vi "Dresden R2R Sputter 03.02.2018 IY24.vi"() -> ()   [LabVIEW 2009] (continued)
                  frame #0 {
                    n3645 = stacked-sequence {
                      frame #0 {
                        n3646 = local write "Pps_code_entry"("PF190=" ("Pps_code_entry")) -> ()
                      }
                      frame #1 {
                        n3647 = Wait (ms)(milliseconds to wait=u32 500) -> ()  [unwired: 1 out]
                      }
                      frame #2 {
                        n3648 = local write "Ppsok"(TRUE ("Ppsok")) -> ()
                      }
                    }
                  }
                  frame #1 {
                    n3649 = stacked-sequence {
                      frame #0 {
                        n3650 = local write "Pps_code_entry"("PF189=" ("Pps_code_entry")) -> ()
                      }
                      frame #1 {
                        n3651 = Wait (ms)(milliseconds to wait=u32 500) -> ()  [unwired: 1 out]
                      }
                      frame #2 {
                        n3652 = local write "Ppsok"(TRUE ("Ppsok")) -> ()
                      }
                    }
                  }
                }
              }
            }
            n3653 = case shown="True" w4784 {
              tunnel: w4788 -> [_ w5137]
              frame #0 {
              }
              frame #1 {
                n3654 = case shown="False" w5137 {
                  frame #0 {
                    n3655 = stacked-sequence {
                      frame #0 {
                        n3656 = local write "Pps_code_entry"("PF220=" ("Pps_code_entry")) -> ()
                      }
                      frame #1 {
                        n3657 = Wait (ms)(milliseconds to wait=u32 500) -> ()  [unwired: 1 out]
                      }
                      frame #2 {
                        n3658 = local write "Ppsok"(TRUE ("Ppsok")) -> ()
                      }
                    }
                  }
                  frame #1 {
                    n3659 = stacked-sequence {
                      frame #0 {
                        n3660 = local write "Pps_code_entry"("PF219=" ("Pps_code_entry")) -> ()
                      }
                      frame #1 {
                        n3661 = Wait (ms)(milliseconds to wait=u32 500) -> ()  [unwired: 1 out]
                      }
                      frame #2 {
                        n3662 = local write "Ppsok"(TRUE ("Ppsok")) -> ()
                      }
                    }
                  }
                }
              }
            }
            n3663 = case shown="True" w4944 {
              tunnel: w4948 -> [_ w5368]
              frame #0 {
              }
              frame #1 {
                n3664 = case shown="True" w5368 {
                  frame #0 {
                    n3665 = stacked-sequence {
                      frame #0 {
                        n3666 = local write "Pps_code_entry"("PF156=" ("Pps_code_entry")) -> ()
                      }
                      frame #1 {
                        n3667 = Wait (ms)(milliseconds to wait=u32 500) -> ()  [unwired: 1 out]
                      }
                      frame #2 {
                        n3668 = local write "Ppsok"(TRUE ("Ppsok")) -> ()
                      }
                    }
                  }
                  frame #1 {
                    n3669 = stacked-sequence {
                      frame #0 {
                        n3670 = local write "Pps_code_entry"("PF155=" ("Pps_code_entry")) -> ()
                      }
                      frame #1 {
                        n3671 = Wait (ms)(milliseconds to wait=u32 500) -> ()  [unwired: 1 out]
                      }
                      frame #2 {
                        n3672 = local write "Ppsok"(TRUE ("Ppsok")) -> ()
                      }
                    }
                  }
                }
              }
            }
            n3673 = case shown="True" w5044 {
              tunnel: w5048 -> [_ w5466]
              frame #0 {
              }
              frame #1 {
                n3674 = case shown="True" w5466 {
                  frame #0 {
                    n3675 = stacked-sequence {
                      frame #0 {
                        n3676 = local write "Pps_code_entry"("PF124=" ("Pps_code_entry")) -> ()
                      }
                      frame #1 {
                        n3677 = Wait (ms)(milliseconds to wait=u32 500) -> ()  [unwired: 1 out]
                      }
                      frame #2 {
                        n3678 = local write "Ppsok"(TRUE ("Ppsok")) -> ()
                      }
                    }
                  }
                  frame #1 {
                    n3679 = stacked-sequence {
                      frame #0 {
                        n3680 = local write "Pps_code_entry"("PF123=" ("Pps_code_entry")) -> ()
                      }
                      frame #1 {
                        n3681 = Wait (ms)(milliseconds to wait=u32 500) -> ()  [unwired: 1 out]
                      }
                      frame #2 {
                        n3682 = local write "Ppsok"(TRUE ("Ppsok")) -> ()
                      }
                    }
                  }
                }
              }
            }
            n3683 = case shown="True" w5053 {
              tunnel: w5049 -> [_ w5473]
              frame #0 {
              }
              frame #1 {
                n3684 = case shown="False" w5473 {
                  frame #0 {
                    n3685 = stacked-sequence {
                      frame #0 {
                        n3686 = local write "Pps_code_entry"("PF122=" ("Pps_code_entry")) -> ()
                      }
                      frame #1 {
                        n3687 = Wait (ms)(milliseconds to wait=u32 500) -> ()  [unwired: 1 out]
                      }
                      frame #2 {
                        n3688 = local write "Ppsok"(TRUE ("Ppsok")) -> ()
                      }
                    }
                  }
                  frame #1 {
                    n3689 = stacked-sequence {
                      frame #0 {
                        n3690 = local write "Pps_code_entry"("PF121=" ("Pps_code_entry")) -> ()
                      }
                      frame #1 {
                        n3691 = Wait (ms)(milliseconds to wait=u32 500) -> ()  [unwired: 1 out]
                      }
                      frame #2 {
                        n3692 = local write "Ppsok"(TRUE ("Ppsok")) -> ()
                      }
                    }
                  }
                }
              }
            }
          }
        }
        n3693 = stacked-sequence {
          frame #0 {
            n3694 = local read "Statue_abort"() -> (w4250:bool)
            n3695 = local read "Semi"() -> (w4246:bool)
            n3696 = feedback #116() -> (w4249:bool)  [unwired: 1 in]
            n3697 = case shown="True" w4250 {
              frame #0 {
              }
              frame #1 {
                n3698 = local write "Semi"(TRUE ("Statue_abort")) -> ()
              }
            }
            n3699 = Boolean To (0,1)(Boolean=w4246) -> (0, 1=w4247:i16)
            n3700 = Boolean To (0,1)(Boolean=w4249) -> (0, 1=w4248:i16)
            n3701 = Greater?(x=w4247, y=w4248) -> (0:w4245:bool)
            n3702 = case shown="True" w4245 {
              frame #0 {
              }
              frame #1 {
                n3703 = property on="Process_flow" class="Str"() -> ("Text.Scroll Position"=w4261:u32)  [unwired: 2 in, 2 out]
                n3704 = Get Date/Time String() -> (date string=w4257:string, time string=w4259:string)  [unwired: 3 in]
                n3705 = local read "Process_flow"() -> (w4252:string)
                n3706 = Add(x=w4261, y=u32 10) -> (x+y=w4262:u32)
                n3707 = Concatenate Strings(w4257, " / " ("string"), w4259) -> (w4256:string)
                n3708 = property on="Process_flow" class="Str"("Text.Scroll Position"=w4262) -> ()  [unwired: 2 in, 2 out]
                n3709 = Concatenate Strings(w4256, "-System was aborted." ("PPSCodeEntry")) -> (w4253:string)
                n3710 = Concatenate Strings(w4252, "\r", w4253) -> (w4251:string)
                n3711 = local write "Process_flow"(w4251) -> ()
              }
            }
          }
        }
        n3712 = case shown="True" "Clear_error" {
          frame #0 {
          }
          frame #1 {
            n3713 = local write "Error Message"("" ("Error Message")) -> ()
          }
        }
        n3714 = stacked-sequence {
          frame #0 {
            w4759 = "." ("string")
            # "Date & Time"
            n3715 = Format Date/Time String(time format string (%c)="%d") -> (date/time string=w4757:string)  [unwired: 2 out]
            n3716 = Format Date/Time String(time format string (%c)="%m") -> (date/time string=w4756:string)  [unwired: 2 out]
            n3717 = Format Date/Time String(time format string (%c)="%Y") -> (date/time string=w4758:string)  [unwired: 2 out]
            n3718 = Format Date/Time String(time format string (%c)="%X") -> (date/time string=w4755:string)  [unwired: 2 in]
            n3719 = Concatenate Strings(w4757, w4759, w4756, w4759, w4758, "     " ("string"), w4755) -> (→"Date_time":string)
          }
        }
        n3720 = stacked-sequence {
          frame #0 {
            n3721 = local read "Ch2_Ch_atm_di"() -> (w4295:bool)
            n3722 = local read "Ch1_Ch_atm_di"() -> (w4296:bool)
            n3723 = local read "Ch2_Pl_atm_di"() -> (w4294:bool)
            n3724 = local read "Ch1_Pl_atm_di"() -> (w4297:bool)
            n3725 = case shown="True" w4295 {
              frame #0 {
              }
              frame #1 {
                n3726 = local write "Ch2_Ch_vbv_do"(FALSE ("Ch1_Pl_atm_do")) -> ()
              }
            }
            n3727 = case shown="True" w4296 {
              frame #0 {
              }
              frame #1 {
                n3728 = local write "Ch1_Ch_vbv_do"(FALSE ("Ch1_Pl_atm_do")) -> ()
              }
            }
            n3729 = case shown="True" w4294 {
              frame #0 {
              }
              frame #1 {
                n3730 = local write "Ch2_Pl_vbv_do"(FALSE ("Ch1_Pl_atm_do")) -> ()
              }
            }
            n3731 = case shown="True" w4297 {
              frame #0 {
              }
              frame #1 {
                n3732 = local write "Ch1_Pl_vbv_do"(FALSE ("Ch1_Pl_atm_do")) -> ()
              }
            }
            n3733 = local read "Ch4_Ch_atm_di"() -> (w4292:bool)
            n3734 = local read "Ch3_Ch_atm_di"() -> (w4291:bool)
            n3735 = local read "Ch4_Pl_atm_di"() -> (w4293:bool)
            n3736 = local read "Ch3_Pl_atm_di"() -> (w4290:bool)
            n3737 = case shown="True" w4292 {
              frame #0 {
              }
              frame #1 {
                n3738 = local write "Ch4_Ch_vbv_do"(FALSE ("Ch1_Pl_atm_do")) -> ()
              }
            }
            n3739 = case shown="True" w4291 {
              frame #0 {
              }
              frame #1 {
                n3740 = local write "Ch3_Ch_vbv_do"(FALSE ("Ch1_Pl_atm_do")) -> ()
              }
            }
            n3741 = case shown="True" w4293 {
              frame #0 {
              }
              frame #1 {
                n3742 = local write "Ch4_Pl_vbv_do"(FALSE ("Ch1_Pl_atm_do")) -> ()
              }
            }
            n3743 = case shown="True" w4290 {
              frame #0 {
              }
              frame #1 {
                n3744 = local write "Ch3_Pl_vbv_do"(FALSE ("Ch1_Pl_atm_do")) -> ()
              }
            }
          }
        }
        n3745 = case shown="True" "Left_Direction" {
          frame #0 {
          }
          frame #1 {
            n3746 = local write "Casette_servo_left_direction_do"(TRUE ("Casette_servo_left_direction_do")) -> ()
          }
        }
        n3747 = case shown="True" "Right_Direction" {
          frame #0 {
          }
          frame #1 {
            n3748 = local write "Casette_servo_left_direction_do"(FALSE ("Casette_servo_left_direction_do")) -> ()
          }
        }
      }
    }
    "Background" <- w1835
  }
  n3749 = call <vilib>:"Read JPEG File.vi"("path to JPEG file"="Background_ch4_front_path") -> ("image data"=w542:T34)  [unwired: 8 in, 2 out]
  n3750 = call <vilib>:"MB Serial Init.vi"("Timeout"=i32? 2000, "Mode"=w22, "Parity"=w20, "Baud Rate"=i32? 9600, "VISA resource name"="Moxa I/O 1") -> ("error out"=w16:errorcluster, "VISA resource name out"=w17:refnum<visa-resource-name>)  [unwired: 2 in, 3 out]
  n3751 = call <vilib>:"Read JPEG File.vi"("path to JPEG file"="Background_ch1_front_path") -> ("image data"=w385:T34)  [unwired: 8 in, 2 out]
  n3752 = call <vilib>:"Read JPEG File.vi"("path to JPEG file"="Background_ch4_top_path") -> ("image data"=w541:T34)  [unwired: 8 in, 2 out]
  n3753 = call <vilib>:"Read JPEG File.vi"("path to JPEG file"="Background_ch1_top_path") -> ("image data"=w386:T34)  [unwired: 8 in, 2 out]
  n3754 = Get Date/Time In Seconds() -> (seconds since 1Jan1904=w9:timestamp)
  n3755 = call <vilib>:"Unflatten Pixmap.vi"("image data"=w542) -> ("24-bit pixmap"=w585:u32[][])  [unwired: 4 in, 6 out]
  n3756 = Random Number (0-1)() -> (number: 0 to 1=w5:dbl)
  n3757 = call <vilib>:"Unflatten Pixmap.vi"("image data"=w385) -> ("24-bit pixmap"=w370:u32[][])  [unwired: 4 in, 6 out]
  n3758 = call <vilib>:"Read JPEG File.vi"("path to JPEG file"="Background_ch3_front_path") -> ("image data"=w503:T34)  [unwired: 8 in, 2 out]
  n3759 = call <vilib>:"Unflatten Pixmap.vi"("image data"=w541) -> ("24-bit pixmap"=w584:u32[][])  [unwired: 4 in, 6 out]
  n3760 = call <vilib>:"Unflatten Pixmap.vi"("image data"=w386) -> ("24-bit pixmap"=w371:u32[][])  [unwired: 4 in, 6 out]
  n3761 = Multiply(x=w5, y=i32? 360 ("milliseconds to wait")) -> (x*y=w3:dbl)
  n3762 = call <vilib>:"Unflatten Pixmap.vi"("image data"=w503) -> ("24-bit pixmap"=w571:u32[][])  [unwired: 4 in, 6 out]
  n3763 = call <vilib>:"Read JPEG File.vi"("path to JPEG file"="Background_ch3_top_path") -> ("image data"=w490:T34)  [unwired: 8 in, 2 out]
  n3764 = Build Path(base path="Gui_ch4_front_path", name or relative path="magnetron on.jpg") -> (appended path=w523:path)
  n3765 = Build Path(base path="Gui_ch4_front_path", name or relative path="gv front open.jpg") -> (appended path=w530:path)
  n3766 = Build Path(base path="Gui_ch4_front_path", name or relative path="gv front failed.jpg") -> (appended path=w529:path)
  n3767 = Build Path(base path="Gui_ch4_front_path", name or relative path="magnetron water cooled on.jpg") -> (appended path=w520:path)
  n3768 = Build Path(base path="Gui_ch4_front_path", name or relative path="magnetron water cooled failed.jpg") -> (appended path=w517:path)
  n3769 = Build Path(base path="Gui_ch1_front_path", name or relative path="magnetron on.jpg") -> (appended path=w404:path)
  n3770 = Build Path(base path="Gui_ch1_front_path", name or relative path="gv front open2.jpg") -> (appended path=w397:path)
  n3771 = Build Path(base path="Gui_ch1_front_path", name or relative path="gv front failled2.jpg") -> (appended path=w398:path)
  n3772 = Build Path(base path="Gui_ch1_front_path", name or relative path="magnetron water cooled on.jpg") -> (appended path=w407:path)
  n3773 = Build Path(base path="Gui_ch4_top_path", name or relative path="bv2 on.jpg") -> (appended path=w313:path)
  n3774 = Build Path(base path="Gui_ch4_top_path", name or relative path="sov on.jpg") -> (appended path=w300:path)
  n3775 = Build Path(base path="Gui_ch1_front_path", name or relative path="magnetron water cooled failed.jpg") -> (appended path=w410:path)
  n3776 = Build Path(base path="Gui_ch4_top_path", name or relative path="bv2 fail.jpg") -> (appended path=w310:path)
  n3777 = Build Path(base path="Gui_ch4_top_path", name or relative path="sov fail.jpg") -> (appended path=w303:path)
  n3778 = Build Path(base path="Gui_ch1_front_path", name or relative path="bv3 fail.jpg") -> (appended path=w106:path)
  n3779 = Build Path(base path="Gui_ch4_front_path", name or relative path="bv2 on.jpg") -> (appended path=w365:path)
  n3780 = Build Path(base path="Gui_ch3_front_path", name or relative path="bv3 fail.jpg") -> (appended path=w149:path)
  n3781 = Build Path(base path="Gui_ch3_front_path", name or relative path="gv front open.jpg") -> (appended path=w473:path)
  n3782 = Build Path(base path="Gui_ch3_front_path", name or relative path="magnetron on.jpg") -> (appended path=w477:path)
  n3783 = Build Path(base path="Gui_ch1_front_path", name or relative path="bv3 on.jpg") -> (appended path=w103:path)
  n3784 = Build Path(base path="Gui_ch4_front_path", name or relative path="chamber front piston open drum failed.jpg") -> (appended path=w537:path)
  n3785 = Build Path(base path="Gui_ch4_front_path", name or relative path="bv2 fail.jpg") -> (appended path=w368:path)
  n3786 = Build Path(base path="Gui_ch3_front_path", name or relative path="chamber front piston open.jpg") -> (appended path=w487:path)
  n3787 = Build Path(base path="Gui_ch3_front_path", name or relative path="gv front failed.jpg") -> (appended path=w474:path)
  n3788 = Build Path(base path="Gui_ch3_front_path", name or relative path="bv3 on.jpg") -> (appended path=w146:path)
  n3789 = Build Path(base path="Gui_ch4_front_path", name or relative path="chamber front piston failed drum open.jpg") -> (appended path=w538:path)
  n3790 = Build Path(base path="Gui_ch4_front_path", name or relative path="chamber front piston open.jpg") -> (appended path=w527:path)
  n3791 = Build Path(base path="Gui_ch3_front_path", name or relative path="chamber front piston open drum failed.jpg") -> (appended path=w499:path)
  n3792 = while {
    shift-right: [w5561] -> _
    shift-left: w2 -> [w5538]
    shift-right: [w5558] -> _
    shift-left: i32? 1 -> [w5549]
    shift-right: [w5551] -> _
    shift-left: data[5B] -> [w5557]
    shift-right: [w5550] -> _
    shift-left: i32? 1 -> [w5555]
    shift-right: [w5547] -> _
    shift-left: data[5B] -> [w5556]
    shift-left: w2 -> [w5537]
    shift-right: [w5553] -> _
    shift-left: w9 -> [w5554]
    shift-right: [w5548] -> _
    shift-left: data[5B] ("array") -> [w5552]
    shift-right: [w5536] -> _
    shift-left: data[5B] -> [w5546]
    shift-right: [w5542] -> _
    shift-left: dbl? 6.85 ("To Left Volt") -> [_]
    shift-left: w2 -> [w5541]
    shift-left: w2 -> [_]
    stop <- w5539 stop-if-true
    n3793 = Divide(x=u32 100 ("millisecond multiple"), y=w5549) -> (x/y=w5559:dbl)
    n3794 = local read "Test_stop"() -> (w5544:bool)
    n3795 = Wait Until Next ms Multiple(millisecond multiple=w5559) -> ()  [unwired: 1 out]
    n3796 = Select(t=Roll_StatusT."Stop" ("Roll Status"), s=w5544, f=w5538) -> (s? t:f=w5545:T1)
    n3797 = case shown="\"Start\"" w5545 {
      tunnel: [Roll_StatusT."Initiate" ("Roll Status") w5594 Roll_StatusT."HomeP" ("Roll Status") w5626 w5659 w5686 w5710 w5781 Roll_StatusT."Initiate" ("Roll Status") Roll_StatusT."Stop" ("Roll Status")] -> w5561
      tunnel: [1 w5593 10 10 10 w5670 w5732 10 1 1] -> w5558
      tunnel: [w5567 "Lap Count" w5613 w5629 w5658 w5667 w5716 w5780 w5808 w5825] -> w5551
      tunnel: w5557 -> [w5567 _ w5613 w5629 w5658 w5683 w5715 w5780 w5808 w5825]
      tunnel: [w5568 "Cycle Sayisi" w5614 w5628 w5657 w5671 w5733 w5765 w5809 w5824] -> w5550
      tunnel: w5556 -> [w5566 w5590 w5612 w5631 w5654 w5677 w5728 w5763 w5807 w5826]
      tunnel: [w5566 w5590 w5612 w5631 w5654 w5678 w5728 w5762 w5807 w5826] -> w5547
      tunnel: w5555 -> [w5568 _ w5614 w5628 w5657 w5671 w5733 w5773 w5809 w5824]
      tunnel: w5537 -> [_ _ _ _ _ _ w5708 _ _ _]
      tunnel: w5554 -> [_ w5588 w5609 _ _ w5676 _ w5772 w5811 w5820]
      tunnel: [w5564 w5588 w5609 w5625 w5655 w5675 w5730 w5771 w5811 w5820] -> w5553
      tunnel: w5552 -> [w5569 w5589 w5610 w5624 w5656 w5672 w5724 w5770 w5812 w5821]
      tunnel: [w5569 w5589 w5610 w5624 w5656 w5673 w5723 w5769 w5813 w5821] -> w5548
      tunnel: w5549 -> [_ _ _ _ _ w5670 w5732 _ _ _]
      tunnel: [w5565 w5583 w5608 w5630 w5651 w5668 w5731 w5766 0 0] -> w5536
      tunnel: w5546 -> [w5565 w5587 w5608 w5630 w5651 w5668 w5731 w5766 _ _]
      tunnel: [w5563 w5584 w5607 w5632 w5649 w5666 w5726 w5761 w5803 w5817] -> w5542
      tunnel: "Speed" -> [w5563 w5584 w5607 w5632 w5649 w5666 w5726 w5761 w5803 w5817]
      tunnel: w5537 -> [_ _ _ _ _ _ w5725 _ _ _]
      tunnel: "Speed" -> [_ _ _ _ _ _ _ _ _ _]
      tunnel: w5541 -> [_ _ _ _ _ _ _ _ _ _]
      frame #0 {
        n3798 = flat-sequence {
          tunnel: [w5579] -> w5562
          tunnel: w5562 -> [w5581]
          frame #0 {
            w5572 = FALSE ("Ch1_Motor_DO")
            n3799 = local write "Ch2_SRV_start_stop_do"(w5572) -> ()
            n3800 = local write "Ch3_SRV_start_stop_do"(w5572) -> ()
            n3801 = local write "Ch4_SRV_start_stop_do"(w5572) -> ()
            n3802 = local write "Ch1_SRV_start_stop_do"(w5572) -> ()
            n3803 = local write "Ch1_Motor_DO"(w5572) -> ()
            n3804 = local write "Ch2_Motor_DO"(w5572) -> ()
            n3805 = local write "Ch3_Motor_DO"(w5572) -> ()
            n3806 = local write "Ch4_Motor_DO"(w5572) -> ()
          }
          frame #1 {
            w5573 = sgl 15.0 ("TC1_set_value")
            n3807 = local write "TC2_set_value"(w5573) -> ()
            n3808 = local write "TC1_set_value"(w5573) -> ()
            n3809 = Wait (ms)(milliseconds to wait=u32 10000) -> ()  [unwired: 1 out]
          }
          frame #2 {
            w5577 = 0.9
            n3810 = local write "To Right Volt"(w5577) -> ()
            n3811 = local write "To Left Volt"(0.9) -> ()
            n3812 = local write "To Left Volt"(w5577) -> ()
            n3813 = local write "TC1_set"(TRUE ("Tension Parametre Set Yolla")) -> ()
          }
          frame #3 {
            w5579 = TRUE ("Tension Parametre Set Yolla")
            n3814 = local write "Parameters_set"(w5579) -> ()
            n3815 = Wait (ms)(milliseconds to wait=u32 10000) -> ()  [unwired: 1 out]
          }
          frame #4 {
            n3816 = local write "Calculate_auto"(w5581) -> ()
            n3817 = Wait (ms)(milliseconds to wait=u32 10000) -> ()  [unwired: 1 out]
          }
        }
        n3818 = Get Date/Time In Seconds() -> (seconds since 1Jan1904=w5564:timestamp)
      }
      frame #1 {
        w5586 = 0.0 ("Forward Time")
        # "Kac metre gidilecek bilgisi alınır\nKac tur atacak bilgisi alınır"
        n3819 = local read "Start_roll"() -> (w5585:bool)
        n3820 = case shown="True" w5585 {
          tunnel: [Roll_StatusT."Initiate" ("Roll Status") w5598] -> w5594
          tunnel: [1 10] -> w5593
          tunnel: w5587 -> [_ w5601]
          frame #0 {
          }
          frame #1 {
            n3821 = Not Equal?(x=w5601, y=0) -> (x != y?=w5599:bool)
            n3822 = Wait (ms)(milliseconds to wait=u32 1000) -> ()  [unwired: 1 out]
            n3823 = Select(t=Roll_StatusT."Start" ("Roll Status"), s=w5599, f=Roll_StatusT."Security" ("Roll Status")) -> (s? t:f=w5598:T1)
          }
        }
        n3824 = local write "Forward Time"(w5586) -> ()
        n3825 = local write "Bacward Time"(w5586) -> ()
        n3826 = local read "ch_present_position"() -> (w5583:dbl)
        n3827 = Decrement(x=w5583) -> (x-1=w5582:dbl)
        n3828 = local write "Target Chamber Sensor"(w5582) -> ()
      }
      frame #2 {
        w5606 = 0.9
        n3829 = case shown="4" w5608 {
          frame #0 {
          }
          frame #1 {
            w5616 = TRUE ("Ch1_Motor_DO")
            n3830 = local write "Ch1_Motor_DO"(w5616) -> ()
            n3831 = local write "Ch1_SRV_start_stop_do"(w5616) -> ()
          }
          frame #2 {
            w5617 = TRUE ("Ch1_Motor_DO")
            n3832 = local write "Ch2_Motor_DO"(w5617) -> ()
            n3833 = local write "Ch2_SRV_start_stop_do"(w5617) -> ()
          }
          frame #3 {
            w5618 = TRUE ("Ch1_Motor_DO")
            n3834 = local write "Ch3_Motor_DO"(w5618) -> ()
            n3835 = local write "Ch3_SRV_start_stop_do"(w5618) -> ()
          }
          frame #4 {
            w5619 = TRUE ("Ch1_Motor_DO")
            n3836 = local write "Ch4_Motor_DO"(w5619) -> ()
            n3837 = local write "Ch4_SRV_start_stop_do"(w5619) -> ()
          }
        }
        n3838 = local write "To Right Volt"(w5606) -> ()
        n3839 = local write "To Left Volt"(0.9) -> ()
        n3840 = local write "To Left Volt"(w5606) -> ()
      }
      frame #3 {
        w5621 = 0.9
        # "Dolu yarim aya girince baslatir."
        n3841 = case shown="1" w5630 {
          tunnel: [FALSE ("Ch4_Sensor_DI") w5639 w5640 w5641 w5642] -> w5635
          frame #0 {
          }
          frame #1 {
            n3842 = local read "Ch1_Sensor_DI"() -> (w5639:bool)
          }
          frame #2 {
            n3843 = local read "Ch2_Sensor_DI"() -> (w5640:bool)
          }
          frame #3 {
            n3844 = local read "Ch3_Sensor_DI"() -> (w5641:bool)
          }
          frame #4 {
            n3845 = local read "Ch4_Sensor_DI"() -> (w5642:bool)
          }
        }
        n3846 = feedback #117(FALSE ("Ch4_Sensor_DI")) -> (w5622:bool)
        n3847 = Not(x=w5635) -> (.not. x?=w5623:bool)
        n3848 = And(x=w5623, y=w5622) -> (x .and. y?=w5637:bool)
        n3849 = local write "To Right Volt"(w5621) -> ()
        n3850 = local write "To Left Volt"(0.9) -> ()
        n3851 = local write "To Left Volt"(w5621) -> ()
        n3852 = Select(t=Roll_StatusT."Pause" ("Roll Status"), s=w5637, f=Roll_StatusT."HomeP" ("Roll Status")) -> (s? t:f=w5626:T1)
        n3853 = Get Date/Time In Seconds() -> (seconds since 1Jan1904=w5625:timestamp)
      }
      frame #4 {
        # "Dolu yarim aya girince baslatir."
        n3854 = case shown="4" w5651 {
          tunnel: [FALSE ("Ch4_Sensor_DI") w5662 w5663 w5664 w5665] -> w5652
          frame #0 {
          }
          frame #1 {
            n3855 = local read "Ch1_Sensor_DI"() -> (w5662:bool)
          }
          frame #2 {
            n3856 = local read "Ch2_Sensor_DI"() -> (w5663:bool)
          }
          frame #3 {
            n3857 = local read "Ch3_Sensor_DI"() -> (w5664:bool)
          }
          frame #4 {
            n3858 = local read "Ch4_Sensor_DI"() -> (w5665:bool)
          }
        }
        n3859 = feedback #118(FALSE ("Ch4_Sensor_DI")) -> (w5645:bool)
        n3860 = Not(x=w5652) -> (.not. x?=w5646:bool)
        n3861 = And(x=w5646, y=w5645) -> (x .and. y?=w5647:bool)
        n3862 = local write "To Left Volt"(0.9) -> ()
        n3863 = local write "To Left Volt"(0.9) -> ()
        n3864 = Select(t=Roll_StatusT."Pause" ("Roll Status"), s=w5647, f=Roll_StatusT."Home" ("Roll Status")) -> (s? t:f=w5659:T1)
        n3865 = Get Date/Time In Seconds() -> (seconds since 1Jan1904=w5655:timestamp)
      }
      frame #5 {
        # "Baslangicta dolu yarim ayda ilerler,\nIlk tur icinde once bosa cikar ve\nDolu yarim aya tekrar girince tur atmis olur."
        # "Turları geriye sarma islemi yapılıyor"
        n3866 = case shown="4" w5668 {
          tunnel: [FALSE ("Ch1_Home_DO") w5691 w5692 w5693 w5694] -> w5669
          frame #0 {
          }
          frame #1 {
            n3867 = local read "Ch1_Sensor_DI"() -> (w5691:bool)
          }
          frame #2 {
            n3868 = local read "Ch2_Sensor_DI"() -> (w5692:bool)
          }
          frame #3 {
            n3869 = local read "Ch3_Sensor_DI"() -> (w5693:bool)
          }
          frame #4 {
            n3870 = local read "Ch4_Sensor_DI"() -> (w5694:bool)
          }
        }
        n3871 = feedback #119(TRUE ("Ch1_Home_DO")) -> (w5689:bool)
        n3872 = Not(x=w5689) -> (.not. x?=w5688:bool)
        n3873 = And(x=w5669, y=w5688) -> (x .and. y?=w5680:bool)
        n3874 = local write "To Left Volt"(w5666) -> ()
        n3875 = local write "To Right Volt"(w5666) -> ()
        n3876 = Increment(x=w5677) -> (x+1=w5679:i32)
        n3877 = Decrement(x=w5683) -> (x-1=w5687:i32)
        n3878 = Select(t=w5679, s=w5680, f=w5677) -> (s? t:f=w5678:i32)
        n3879 = Select(t=w5687, s=w5680, f=w5683) -> (s? t:f=w5667:i32)
        n3880 = Less Or Equal?(x=w5667, y=0) -> (x <= y?=w5674:bool)
        n3881 = Select(t=Roll_StatusT."Pause" ("Roll Status"), s=w5674, f=Roll_StatusT."Forward" ("Roll Status")) -> (s? t:f=w5686:T1)
        n3882 = case shown="False" w5674 {
          tunnel: [w5697 w5702] -> w5675
          tunnel: w5676 -> [w5697 _]
          tunnel: [w5695 w5699] -> w5673
          tunnel: w5672 -> [w5695 w5701]
          frame #0 {
            n3883 = Get Date/Time In Seconds() -> (seconds since 1Jan1904=w5698:timestamp)
            n3884 = Subtract(x=w5698, y=w5697) -> (x-y=→"Forward Time":dbl)
          }
          frame #1 {
            n3885 = local read "Forward Time"() -> (w5700:dbl)
            n3886 = Get Date/Time In Seconds() -> (seconds since 1Jan1904=w5702:timestamp)
            n3887 = Build Array (concatenate)(w5701, w5700) -> (w5699:dbl[])
          }
        }
      }
      frame #6 {
        w5703 = 0.9 ("To Left Volt")
        w5729 = 0.0 ("milliseconds to wait")
        n3888 = flat-sequence {
          tunnel: w5725 -> [w5739]
          tunnel: [w5748] -> w5727
          tunnel: w5727 -> [w5751]
          tunnel: w5731 -> [w5755]
          tunnel: [w5754] -> w5730
          frame #0 {
            w5734 = FALSE ("Ch1_Motor_DO")
            n3889 = local write "Ch2_SRV_start_stop_do"(w5734) -> ()
            n3890 = local write "Ch3_SRV_start_stop_do"(w5734) -> ()
            n3891 = local write "Ch4_SRV_start_stop_do"(w5734) -> ()
            n3892 = local write "Ch1_SRV_start_stop_do"(w5734) -> ()
            n3893 = local write "Ch1_Motor_DO"(w5734) -> ()
            n3894 = local write "Ch2_Motor_DO"(w5734) -> ()
            n3895 = local write "Ch3_Motor_DO"(w5734) -> ()
            n3896 = local write "Ch4_Motor_DO"(w5734) -> ()
            n3897 = local write "Start_roll"(FALSE ("Start")) -> ()
          }
          frame #1 {
            n3898 = Equal?(x=Roll_StatusT."Backward" ("Roll Status"), y=w5739) -> (x = y?=w5740:bool)
            n3899 = Equal?(x=Roll_StatusT."Home" ("Roll Status"), y=w5739) -> (x = y?=w5737:bool)
            n3900 = Or(x=w5737, y=w5740) -> (x .or. y?=w5736:bool)
            n3901 = case shown="False" w5736 {
              frame #0 {
                n3902 = local read "Roll_side_select"() -> (w5744:enum32{"Left to Right", "Right to Left"})
                n3903 = Equal?(x=enum32{"Left to Right", "Right to Left"}."Left to Right" ("Roll_side_select"), y=w5744) -> (x = y?=w5745:bool)
                n3904 = case shown="True" w5745 {
                  frame #0 {
                    n3905 = local write "Roll_side_select"(enum32{"Left to Right", "Right to Left"}."Left to Right" ("Roll_side_select")) -> ()
                  }
                  frame #1 {
                    n3906 = local write "Roll_side_select"(enum32{"Left to Right", "Right to Left"}."Right to Left" ("Roll_side_select")) -> ()
                  }
                }
              }
              frame #1 {
              }
            }
            n3907 = Wait (ms)(milliseconds to wait=u32 1000) -> ()  [unwired: 1 out]
          }
          frame #2 {
            w5748 = TRUE ("Tension Parametre Set Yolla")
            n3908 = local write "Tension Parametre Set"(w5748) -> ()
            n3909 = local write "Parameters_set"(w5748) -> ()
            n3910 = Wait (ms)(milliseconds to wait=u32 5000) -> ()  [unwired: 1 out]
          }
          frame #3 {
            n3911 = local write "Calculate_auto"(w5751) -> ()
            n3912 = Wait (ms)(milliseconds to wait=u32 5000) -> ()  [unwired: 1 out]
          }
          frame #4 {
            n3913 = local write "Start_roll"(TRUE ("Start")) -> ()
            n3914 = Wait (ms)(milliseconds to wait=u32 1000) -> ()  [unwired: 1 out]
          }
          frame #5 {
            n3915 = case shown="4" w5755 {
              frame #0 {
              }
              frame #1 {
                w5756 = TRUE ("Ch1_Motor_DO")
                n3916 = local write "Ch1_SRV_start_stop_do"(w5756) -> ()
                n3917 = local write "Ch1_Motor_DO"(w5756) -> ()
              }
              frame #2 {
                w5757 = TRUE ("Ch1_Motor_DO")
                n3918 = local write "Ch2_SRV_start_stop_do"(w5757) -> ()
                n3919 = local write "Ch2_Motor_DO"(w5757) -> ()
              }
              frame #3 {
                w5758 = TRUE ("Ch1_Motor_DO")
                n3920 = local write "Ch3_SRV_start_stop_do"(w5758) -> ()
                n3921 = local write "Ch3_Motor_DO"(w5758) -> ()
              }
              frame #4 {
                w5759 = TRUE ("Ch1_Motor_DO")
                n3922 = local write "Ch4_SRV_start_stop_do"(w5759) -> ()
                n3923 = local write "Ch4_Motor_DO"(w5759) -> ()
              }
            }
            n3924 = Get Date/Time In Seconds() -> (seconds since 1Jan1904=w5754:timestamp)
          }
        }
        n3925 = Equal?(x=Roll_StatusT."Forward" ("Roll Status"), y=w5708) -> (x = y?=w5717:bool)
        n3926 = Equal?(x=Roll_StatusT."Backward" ("Roll Status"), y=w5708) -> (x = y?=w5707:bool)
        n3927 = Select(t=Roll_StatusT."HomeP" ("Roll Status"), s=w5707, f=Roll_StatusT."Forward" ("Roll Status")) -> (s? t:f=w5705:T1)
        n3928 = local write "To Right Volt"(w5703) -> ()
        n3929 = local write "To Left Volt"(w5703) -> ()
        n3930 = local read "Lap Count"() -> (w5720:i32)
        n3931 = Increment(x=w5720) -> (x+1=w5719:i32)
        n3932 = Select(t=Roll_StatusT."Backward" ("Roll Status"), s=w5717, f=w5705) -> (s? t:f=w5711:T1)
        n3933 = Build Array (concatenate)(w5724, u32 0 ("milliseconds to wait")) -> (w5723:dbl[])
        n3934 = Select(t=w5715, s=w5717, f=w5719) -> (s? t:f=w5716:i32)
        n3935 = local write "Bacward Time"(w5729) -> ()
        n3936 = local write "Forward Time"(w5729) -> ()
        n3937 = Equal?(x=Roll_StatusT."HomeP" ("Roll Status"), y=w5708) -> (x = y?=w5713:bool)
        n3938 = Select(t=Roll_StatusT."Home" ("Roll Status"), s=w5713, f=w5711) -> (s? t:f=w5710:T1)
      }
      frame #7 {
        n3939 = case shown="1" w5766 {
          tunnel: [FALSE ("Ch1_Home_DO") w5789 w5790 w5791 w5792] -> w5767
          frame #0 {
          }
          frame #1 {
            n3940 = local read "Ch1_Sensor_DI"() -> (w5789:bool)
          }
          frame #2 {
            n3941 = local read "Ch2_Sensor_DI"() -> (w5790:bool)
          }
          frame #3 {
            n3942 = local read "Ch3_Sensor_DI"() -> (w5791:bool)
          }
          frame #4 {
            n3943 = local read "Ch4_Sensor_DI"() -> (w5792:bool)
          }
        }
        n3944 = Decrement(x=w5773) -> (x-1=w5779:i32)
        n3945 = feedback #120(TRUE ("Ch1_Home_DO")) -> (w5764:bool)
        n3946 = local write "To Right Volt"(w5761) -> ()
        n3947 = local write "To Left Volt"(w5761) -> ()
        n3948 = Not(x=w5767) -> (.not. x?=w5784:bool)
        n3949 = And(x=w5784, y=w5764) -> (x .and. y?=w5787:bool)
        n3950 = Decrement(x=w5763) -> (x-1=w5786:i32)
        n3951 = Select(t=w5786, s=w5787, f=w5763) -> (s? t:f=w5762:i32)
        n3952 = Less Or Equal?(x=w5762, y=0) -> (x <= y?=w5760:bool)
        n3953 = Select(t=w5779, s=w5760, f=w5773) -> (s? t:f=w5765:i32)
        n3954 = Less Or Equal?(x=w5765, y=0) -> (x <= y?=w5778:bool)
        n3955 = Select(t=Roll_StatusT."Stop" ("Roll Status"), s=w5778, f=Roll_StatusT."Pause" ("Roll Status")) -> (s? t:f=w5774:T1)
        n3956 = Select(t=w5774, s=w5760, f=Roll_StatusT."Backward" ("Roll Status")) -> (s? t:f=w5781:T1)
        n3957 = case shown="True" w5760 {
          tunnel: [w5796 w5801] -> w5771
          tunnel: w5772 -> [w5796 _]
          tunnel: w5770 -> [w5794 w5799]
          tunnel: [w5794 w5800] -> w5769
          frame #0 {
            n3958 = Get Date/Time In Seconds() -> (seconds since 1Jan1904=w5797:timestamp)
            n3959 = Subtract(x=w5797, y=w5796) -> (x-y=w5795:dbl)
            n3960 = Negate(x=w5795) -> (-x=→"Bacward Time":dbl)
          }
          frame #1 {
            n3961 = local read "Bacward Time"() -> (w5798:dbl)
            n3962 = Get Date/Time In Seconds() -> (seconds since 1Jan1904=w5801:timestamp)
            n3963 = Build Array (concatenate)(w5799, w5798) -> (w5800:dbl[])
          }
        }
      }
      frame #8 {
        w5802 = FALSE ("Ch1_Motor_DO")
        n3964 = Wait (ms)(milliseconds to wait=u32 1000) -> ()  [unwired: 1 out]
        n3965 = local write "Start_roll"(FALSE ("Start")) -> ()
        n3966 = local write "Ch1_Motor_DO"(w5802) -> ()
        n3967 = local write "Ch2_Motor_DO"(w5802) -> ()
        n3968 = local write "Ch3_Motor_DO"(w5802) -> ()
        n3969 = local write "Ch4_Motor_DO"(w5802) -> ()
        n3970 = local write "Ch1_SRV_start_stop_do"(w5802) -> ()
        n3971 = local write "Ch2_SRV_start_stop_do"(w5802) -> ()
        n3972 = local write "Ch3_SRV_start_stop_do"(w5802) -> ()
        n3973 = local write "Ch4_SRV_start_stop_do"(w5802) -> ()
        n3974 = Build Array (concatenate)(w5812, u32 0 ("milliseconds to wait")) -> (w5813:dbl[])
      }
      frame #9 {
        w5816 = FALSE ("Ch1_Motor_DO")
        n3975 = local write "Ch1_Motor_DO"(w5816) -> ()
        n3976 = local write "Ch2_Motor_DO"(w5816) -> ()
        n3977 = local write "Ch3_Motor_DO"(w5816) -> ()
        n3978 = local write "Ch4_Motor_DO"(w5816) -> ()
        n3979 = local write "Ch1_SRV_start_stop_do"(w5816) -> ()
        n3980 = local write "Ch2_SRV_start_stop_do"(w5816) -> ()
        n3981 = local write "Ch3_SRV_start_stop_do"(w5816) -> ()
        n3982 = local write "Ch4_SRV_start_stop_do"(w5816) -> ()
        n3983 = local write "Start_roll"(FALSE ("Start")) -> ()
      }
    }
    "Current Forward Lap" <- w5551
    "Current Cycle" <- w5550
    "Lap Times" <- w5548
    "Current Backward Lap" <- w5547
    "Current Chamber" <- w5536
    n3984 = local read "Test_stop"() -> (w5539:bool)
    "Roll Status" <- w5538
  }
  n3985 = Build Path(base path="Gui_ch3_front_path", name or relative path="chamber front piston failed drum open.jpg") -> (appended path=w500:path)
  n3986 = Build Path(base path="Gui_ch3_front_path", name or relative path="magnetron water cooled on.jpg") -> (appended path=w480:path)
  n3987 = Build Path(base path="Gui_ch3_front_path", name or relative path="magnetron water cooled failed.jpg") -> (appended path=w483:path)
  n3988 = Build Path(base path="Gui_ch1_front_path", name or relative path="chamber front piston open drum failed.jpg") -> (appended path=w390:path)
  n3989 = Build Path(base path="Gui_ch1_front_path", name or relative path="chamber front piston failed drum open.jpg") -> (appended path=w389:path)
  n3990 = Build Path(base path="Gui_ch1_front_path", name or relative path="chamber front piston open.jpg") -> (appended path=w400:path)
  n3991 = Build Path(base path="Gui_ch3_front_path", name or relative path="gv front failled2.jpg") -> (appended path=w359:path)
  n3992 = Build Path(base path="Gui_ch3_front_path", name or relative path="gv front open2.jpg") -> (appended path=w356:path)
  n3993 = call <vilib>:"Read JPEG File.vi"("path to JPEG file"="Background_ch2_front_path") -> ("image data"=w463:T34)  [unwired: 8 in, 2 out]
  n3994 = Build Path(base path="Gui_ch2_top_path", name or relative path="bv2 on.jpg") -> (appended path=w276:path)
  n3995 = Build Path(base path="Gui_ch4_top_path", name or relative path="chamber 1 top piston open.jpg") -> (appended path=w512:path)
  n3996 = call <vilib>:"Unflatten Pixmap.vi"("image data"=w490) -> ("24-bit pixmap"=w566:u32[][])  [unwired: 4 in, 6 out]
  n3997 = Build Path(base path="Gui_ch2_top_path", name or relative path="sov on.jpg") -> (appended path=w286:path)
  n3998 = Build Path(base path="Gui_ch4_top_path", name or relative path="chamber 1 top piston failed.jpg") -> (appended path=w511:path)
  n3999 = Build Path(base path="Gui_ch2_top_path", name or relative path="bv2 fail.jpg") -> (appended path=w279:path)
  n4000 = Build Path(base path="Gui_ch4_top_path", name or relative path="atm3 fail.jpg") -> (appended path=w349:path)
  n4001 = Build Path(base path="Gui_ch2_top_path", name or relative path="sov fail.jpg") -> (appended path=w283:path)
  n4002 = Build Path(base path="Gui_ch2_front_path", name or relative path="gv front open.jpg") -> (appended path=w456:path)
  n4003 = Build Path(base path="Gui_ch2_front_path", name or relative path="magnetron on.jpg") -> (appended path=w452:path)
  n4004 = Build Path(base path="Gui_ch4_top_path", name or relative path="atm3 on.jpg") -> (appended path=w348:path)
  n4005 = Build Path(base path="Gui_ch4_top_path", name or relative path="pg2 fail.jpg") -> (appended path=w340:path)
  n4006 = Build Path(base path="Gui_ch4_top_path", name or relative path="cc fail.jpg") -> (appended path=w333:path)
  n4007 = Build Path(base path="Gui_ch4_top_path", name or relative path="pg2 fail.jpg") -> (appended path=w325:path)
  n4008 = Build Path(base path="Gui_ch2_top_path", name or relative path="bv3 fail.jpg") -> (appended path=w155:path)
  n4009 = Build Path(base path="Gui_ch2_front_path", name or relative path="chamber front piston open.jpg") -> (appended path=w444:path)
  n4010 = Build Path(base path="Gui_ch2_front_path", name or relative path="gv front failed.jpg") -> (appended path=w455:path)
  n4011 = Build Path(base path="Gui_ch2_top_path", name or relative path="bv2 on.jpg") -> (appended path=w193:path)
  n4012 = Build Path(base path="Gui_ch4_top_path", name or relative path="pg2 on.jpg") -> (appended path=w341:path)
  n4013 = Build Path(base path="Gui_ch4_top_path", name or relative path="cc on.jpg") -> (appended path=w332:path)
  n4014 = Build Path(base path="Gui_ch4_top_path", name or relative path="pg2 on.jpg") -> (appended path=w324:path)
  n4015 = Build Path(base path="Gui_ch2_front_path", name or relative path="chamber front piston open drum failed.jpg") -> (appended path=w438:path)
  n4016 = Build Path(base path="Gui_ch2_top_path", name or relative path="sov on.jpg") -> (appended path=w183:path)
  n4017 = Build Path(base path="Gui_ch4_top_path", name or relative path="bv1 fail.jpg") -> (appended path=w318:path)
  n4018 = Build Path(base path="Gui_ch2_top_path", name or relative path="bv3 on.jpg") -> (appended path=w158:path)
  n4019 = Build Path(base path="Gui_ch2_front_path", name or relative path="chamber front piston failed drum open.jpg") -> (appended path=w437:path)
  n4020 = Build Path(base path="Gui_ch2_front_path", name or relative path="magnetron water cooled on.jpg") -> (appended path=w449:path)
  n4021 = Build Path(base path="Gui_ch2_top_path", name or relative path="bv2 fail.jpg") -> (appended path=w190:path)
  n4022 = Build Path(base path="Gui_ch4_top_path", name or relative path="gv top open.jpg") -> (appended path=w507:path)
  n4023 = Build Path(base path="Gui_ch4_top_path", name or relative path="bv1 on.jpg") -> (appended path=w319:path)
  n4024 = Build Path(base path="Gui_ch2_top_path", name or relative path="sov fail.jpg") -> (appended path=w186:path)
  n4025 = Build Path(base path="Gui_ch4_top_path", name or relative path="gv top failed.jpg") -> (appended path=w508:path)
  n4026 = Build Path(base path="Gui_ch2_front_path", name or relative path="magnetron water cooled failed.jpg") -> (appended path=w446:path)
  n4027 = Build Path(base path="Gui_ch3_front_path", name or relative path="bv2 on.jpg") -> (appended path=w141:path)
  n4028 = Build Path(base path="Gui_ch3_front_path", name or relative path="bv2 fail.jpg") -> (appended path=w140:path)
  n4029 = Build Path(base path="Gui_ch2_top_path", name or relative path="bv3 fail.jpg") -> (appended path=w129:path)
  n4030 = Build Path(base path="Gui_ch2_top_path", name or relative path="bv3 on.jpg") -> (appended path=w132:path)
  n4031 = call <vilib>:"Read JPEG File.vi"("path to JPEG file"=w523) -> ("image data"=w522:T34)  [unwired: 8 in, 2 out]
  n4032 = call <vilib>:"Read JPEG File.vi"("path to JPEG file"=w530) -> ("image data"=w531:T34)  [unwired: 8 in, 2 out]
  n4033 = call <vilib>:"Read JPEG File.vi"("path to JPEG file"=w529) -> ("image data"=w528:T34)  [unwired: 8 in, 2 out]
  n4034 = call <vilib>:"Read JPEG File.vi"("path to JPEG file"=w520) -> ("image data"=w521:T34)  [unwired: 8 in, 2 out]
  n4035 = call <vilib>:"Read JPEG File.vi"("path to JPEG file"=w517) -> ("image data"=w516:T34)  [unwired: 8 in, 2 out]
  n4036 = call <vilib>:"Read JPEG File.vi"("path to JPEG file"=w404) -> ("image data"=w405:T34)  [unwired: 8 in, 2 out]
  n4037 = while {
    shift-right: [w5828] -> _
    shift-left: w3 -> [w5831]
    stop <- w5829 continue-if-true
    w5830 = u32 10 ("milliseconds to wait")
    n4038 = Wait (ms)(milliseconds to wait=w5830) -> ()  [unwired: 1 out]
    n4039 = In Range and Coerce(upper limit=270, x=w5831, lower limit=90) -> (In Range?=w5827:bool)  [unwired: 1 out]
    n4040 = local read "Ch1_Motor_DO"() -> (w5834:bool)
    n4041 = local write "Sensor_DI Sim"(w5827) -> ()
    n4042 = case shown="True" w5834 {